vi "Dresden R2R Sputter 03.02.2018 IY24.vi"() -> ()   [LabVIEW 2009] (continued)
                                frame #0 {
                                n26763 = while {
                                i -> [w31945]
                                stop <- w31941 stop-if-true
                                n26764 = local read "Pc_bv_opened_ch3"() -> (w31943:bool)
                                n26765 = Greater?(x=w31945, y=120) -> (0:w31944:bool)
                                n26766 = local read "Semi"() -> (w31942:bool)
                                n26767 = Compound Arithmetic op=OR(w31942, w31943, w31944) -> (w31941:bool)
                                n26768 = Wait (ms)(milliseconds to wait=u32 500) -> ()  [unwired: 1 out]
                                }
                                }
                                frame #1 {
                                }
                                }
                                }
                                frame #6 {
                                n26769 = local read "Semi"() -> (w31947:bool)
                                n26770 = case shown="False" w31947 {
                                frame #0 {
                                n26771 = local read "Pc_bv_opened_ch3"() -> (w31948:bool)
                                n26772 = case shown="False" w31948 {
                                frame #0 {
                                n26773 = local write "Error Message"("Start up process  cancelled\nbecause  PC-BV not opened.\nPlease check PC-BV1 connections." ("Error Message")) -> ()
                                n26774 = Wait (ms)(milliseconds to wait=u32 1000) -> ()  [unwired: 1 out]
                                }
                                frame #1 {
                                }
                                }
                                }
                                frame #1 {
                                }
                                }
                                }
                                }
                                }
                                frame #1 {
                                }
                                }
                                }
                                frame #1 {
                                n26775 = local read "Semi"() -> (w31951:bool)
                                n26776 = case shown="False" w31951 {
                                frame #0 {
                                n26777 = Wait (ms)(milliseconds to wait=u32 1000) -> ()  [unwired: 1 out]
                                n26778 = local write "SDC1 7"(TRUE ("SDC1 7")) -> ()
                                }
                                frame #1 {
                                }
                                }
                                }
                                }
                                }
                                frame #10 {
                                # "CC OPEN"
                                n26779 = stacked-sequence {
                                frame #0 {
                                n26780 = local read "Semi"() -> (w31954:bool)
                                n26781 = case shown="False" w31954 {
                                frame #0 {
                                n26782 = while {
                                i -> [w31960]
                                stop <- w31955 stop-if-true
                                n26783 = Greater?(x=w31960, y=50) -> (0:w31959:bool)
                                n26784 = case shown="True" w31959 {
                                frame #0 {
                                }
                                frame #1 {
                                n26785 = local write "Semi"(TRUE ("Semi")) -> ()
                                n26786 = local write "Error Message"("Coating Process  \nwas cancelled.\nPlease check \nBG-BV connection." ("Error Message")) -> ()
                                }
                                }
                                n26787 = local read "Ch3_Cc_on_off_di"() -> (w31958:bool)
                                n26788 = case shown="False" w31958 {
                                tunnel: [FALSE TRUE] -> w31957
                                frame #0 {
                                n26789 = local write "Ch3_Cc_on_off_do"(TRUE ("Ch1_WFC_do")) -> ()
                                n26790 = Wait Until Next ms Multiple(millisecond multiple=u32 200) -> ()  [unwired: 1 out]
                                }
                                frame #1 {
                                }
                                }
                                n26791 = local read "Semi"() -> (w31956:bool)
                                n26792 = Or(x=w31957, y=w31956) -> (x .or. y?=w31955:bool)
                                }
                                }
                                frame #1 {
                                }
                                }
                                }
                                frame #1 {
                                n26793 = local read "Semi"() -> (w31968:bool)
                                n26794 = case shown="False" w31968 {
                                frame #0 {
                                n26795 = while {
                                i -> [w31973]
                                stop <- w31971 stop-if-true
                                n26796 = Greater?(x=w31973, y=30) -> (0:w31969:bool)
                                n26797 = Wait Until Next ms Multiple(millisecond multiple=u32 1000) -> ()  [unwired: 1 out]
                                n26798 = local read "Semi"() -> (w31972:bool)
                                n26799 = Or(x=w31969, y=w31972) -> (x .or. y?=w31971:bool)
                                }
                                }
                                frame #1 {
                                }
                                }
                                }
                                frame #2 {
                                n26800 = local read "Semi"() -> (w31975:bool)
                                n26801 = case shown="False" w31975 {
                                frame #0 {
                                n26802 = Wait (ms)(milliseconds to wait=u32 1000) -> ()  [unwired: 1 out]
                                n26803 = local write "SDC1 7b"(TRUE ("SDC1 3")) -> ()
                                }
                                frame #1 {
                                }
                                }
                                }
                                }
                                }
                                frame #11 {
                                # "CHECK CHAMBER PRESSURE"
                                n26804 = stacked-sequence {
                                frame #0 {
                                n26805 = local read "Semi"() -> (w31978:bool)
                                n26806 = case shown="False" w31978 {
                                frame #0 {
                                n26807 = while {
                                i -> [w31986]
                                stop <- w31980 stop-if-true
                                n26808 = Greater?(x=w31986, y=300) -> (0:w31985:bool)
                                n26809 = case shown="True" w31985 {
                                frame #0 {
                                }
                                frame #1 {
                                n26810 = local write "Semi"(TRUE ("Semi")) -> ()
                                n26811 = local write "Error Message"("Coating Process cancelled.\nPlease check chamber \nconnections." ("Error Message")) -> ()
                                }
                                }
                                n26812 = local read "Ch_CC_press_ch3 2"() -> (w31979:dbl)
                                n26813 = Greater Or Equal?(x=w31979, y=5e-05 ("CHAMBER PRESSURE 5")) -> (x >= y?=w31983:bool)
                                n26814 = case shown="True" w31983 {
                                tunnel: [TRUE FALSE] -> w31982
                                frame #0 {
                                }
                                frame #1 {
                                n26815 = Wait Until Next ms Multiple(millisecond multiple=u32 200) -> ()  [unwired: 1 out]
                                }
                                }
                                n26816 = local read "Semi"() -> (w31981:bool)
                                n26817 = Or(x=w31982, y=w31981) -> (x .or. y?=w31980:bool)
                                }
                                }
                                frame #1 {
                                }
                                }
                                }
                                frame #1 {
                                n26818 = local read "Semi"() -> (w31993:bool)
                                n26819 = case shown="False" w31993 {
                                frame #0 {
                                n26820 = Wait (ms)(milliseconds to wait=u32 1000) -> ()  [unwired: 1 out]
                                n26821 = local write "SDC1 10"(TRUE ("SDC1 10")) -> ()
                                }
                                frame #1 {
                                }
                                }
                                }
                                }
                                }
                                frame #12 {
                                # "CC CLOSE"
                                n26822 = stacked-sequence {
                                frame #0 {
                                n26823 = local read "Semi"() -> (w31996:bool)
                                n26824 = case shown="False" w31996 {
                                frame #0 {
                                n26825 = while {
                                i -> [w32002]
                                stop <- w31997 stop-if-true
                                n26826 = Greater?(x=w32002, y=50) -> (0:w32001:bool)
                                n26827 = case shown="True" w32001 {
                                frame #0 {
                                }
                                frame #1 {
                                n26828 = local write "Semi"(TRUE ("Semi")) -> ()
                                n26829 = local write "Error Message"("Coating Process  \nwas cancelled.\nPlease check \nBG-BV connection." ("Error Message")) -> ()
                                }
                                }
                                n26830 = local read "Ch3_Cc_on_off_di"() -> (w32000:bool)
                                n26831 = case shown="True" w32000 {
                                tunnel: [TRUE FALSE] -> w31999
                                frame #0 {
                                }
                                frame #1 {
                                n26832 = local write "Ch3_Cc_on_off_do"(FALSE ("Ch1_WFC_do")) -> ()
                                n26833 = Wait Until Next ms Multiple(millisecond multiple=u32 200) -> ()  [unwired: 1 out]
                                }
                                }
                                n26834 = local read "Semi"() -> (w31998:bool)
                                n26835 = Or(x=w31999, y=w31998) -> (x .or. y?=w31997:bool)
                                }
                                }
                                frame #1 {
                                }
                                }
                                }
                                frame #1 {
                                n26836 = local read "Semi"() -> (w32010:bool)
                                n26837 = case shown="False" w32010 {
                                frame #0 {
                                n26838 = local write "SDC1 10b"(TRUE ("SDC1 3")) -> ()
                                n26839 = Wait (ms)(milliseconds to wait=u32 1000) -> ()  [unwired: 1 out]
                                }
                                frame #1 {
                                }
                                }
                                }
                                }
                                }
                                frame #13 {
                                # "SET Ar FLOW"
                                n26840 = local read "R_Web_selection"() -> (w32013:enum32{"Web", "Other"})
                                n26841 = case shown="\"Other\"" w32013 {
                                frame #0 {
                                }
                                frame #1 {
                                n26842 = stacked-sequence {
                                frame #0 {
                                n26843 = local read "Semi"() -> (w32014:bool)
                                n26844 = case shown="False" w32014 {
                                frame #0 {
                                n26845 = stacked-sequence {
                                frame #0 {
                                n26846 = local read "Semi"() -> (w32015:bool)
                                n26847 = case shown="False" w32015 {
                                frame #0 {
                                n26848 = local read "R Argon Flow sccm"() -> (w32016:dbl)
                                n26849 = local write "Ar_sccm3_4"(w32016) -> ()
                                }
                                frame #1 {
                                }
                                }
                                }
                                frame #1 {
                                n26850 = local read "Semi"() -> (w32017:bool)
                                n26851 = case shown="False" w32017 {
                                frame #0 {
                                n26852 = local write "Mfc2_Ar _3_4_set"(TRUE ("Mfc_Ar _1_2_set")) -> ()
                                }
                                frame #1 {
                                }
                                }
                                }
                                frame #2 {
                                n26853 = local read "Semi"() -> (w32019:bool)
                                n26854 = case shown="False" w32019 {
                                frame #0 {
                                n26855 = while {
                                i -> [w32022]
                                stop <- w32024 stop-if-true
                                n26856 = Greater?(x=w32022, y=50) -> (0:w32021:bool)
                                n26857 = local read "Semi"() -> (w32020:bool)
                                n26858 = Or(x=w32020, y=w32021) -> (x .or. y?=w32024:bool)
                                }
                                }
                                frame #1 {
                                }
                                }
                                }
                                frame #3 {
                                n26859 = local read "Semi"() -> (w32025:bool)
                                n26860 = case shown="False" w32025 {
                                frame #0 {
                                n26861 = local read "Ar_sccm_act 2"() -> (w32026:dbl)
                                n26862 = Greater?(x=w32026, y=1) -> (0:w32027:bool)
                                n26863 = case shown="False" w32027 {
                                frame #0 {
                                n26864 = local read "R Argon Flow sccm"() -> (w32029:dbl)
                                n26865 = local write "Ar_sccm3_4"(w32029) -> ()
                                }
                                frame #1 {
                                }
                                }
                                }
                                frame #1 {
                                }
                                }
                                }
                                frame #4 {
                                n26866 = local read "Semi"() -> (w32030:bool)
                                n26867 = case shown="False" w32030 {
                                frame #0 {
                                n26868 = local read "Ar_sccm_act 2"() -> (w32031:dbl)
                                n26869 = Greater?(x=w32031, y=1) -> (0:w32032:bool)
                                n26870 = case shown="False" w32032 {
                                frame #0 {
                                n26871 = while {
                                i -> [w32035]
                                stop <- w32039 stop-if-true
                                n26872 = Greater?(x=w32035, y=50) -> (0:w32034:bool)
                                n26873 = local read "Semi"() -> (w32038:bool)
                                n26874 = case shown="False" w32038 {
                                tunnel: [FALSE TRUE] -> w32037
                                frame #0 {
                                n26875 = Wait Until Next ms Multiple(millisecond multiple=u32 200) -> ()  [unwired: 1 out]
                                }
                                frame #1 {
                                }
                                }
                                n26876 = Or(x=w32037, y=w32034) -> (x .or. y?=w32039:bool)
                                }
                                }
                                frame #1 {
                                }
                                }
                                }
                                frame #1 {
                                }
                                }
                                }
                                frame #5 {
                                n26877 = local read "Semi"() -> (w32043:bool)
                                n26878 = case shown="False" w32043 {
                                frame #0 {
                                n26879 = local read "Ar_sccm_act 2"() -> (w32044:dbl)
                                n26880 = Greater?(x=w32044, y=1) -> (0:w32045:bool)
                                n26881 = case shown="False" w32045 {
                                frame #0 {
                                n26882 = local write "Semi"(TRUE ("Semi")) -> ()
                                n26883 = local write "Error Message"("Coating process cancelled.\nPlease check connections." ("Error Message")) -> ()
                                }
                                frame #1 {
                                }
                                }
                                }
                                frame #1 {
                                }
                                }
                                }
                                }
                                }
                                frame #1 {
                                }
                                }
                                }
                                frame #1 {
                                n26884 = local read "Semi"() -> (w32049:bool)
                                n26885 = case shown="False" w32049 {
                                frame #0 {
                                n26886 = local write "SDC1 11"(TRUE ("SDC1 11")) -> ()
                                n26887 = Wait (ms)(milliseconds to wait=u32 1000) -> ()  [unwired: 1 out]
                                }
                                frame #1 {
                                }
                                }
                                }
                                }
                                }
                                }
                                }
                                frame #14 {
                                # "Set  Pressure"
                                n26888 = local read "R_Web_selection"() -> (w32052:enum32{"Web", "Other"})
                                n26889 = case shown="\"Other\"" w32052 {
                                frame #0 {
                                }
                                frame #1 {
                                n26890 = stacked-sequence {
                                frame #0 {
                                n26891 = local read "Semi"() -> (w32053:bool)
                                n26892 = case shown="False" w32053 {
                                frame #0 {
                                n26893 = stacked-sequence {
                                frame #0 {
                                n26894 = local read "Semi"() -> (w32054:bool)
                                n26895 = case shown="False" w32054 {
                                frame #0 {
                                n26896 = local read "R Set Pressure mtorr"() -> (w32055:dbl)
                                n26897 = local write "Set_pressure_value 3"(w32055) -> ()
                                }
                                frame #1 {
                                }
                                }
                                }
                                frame #1 {
                                n26898 = local read "Semi"() -> (w32056:bool)
                                n26899 = case shown="False" w32056 {
                                frame #0 {
                                n26900 = Wait (ms)(milliseconds to wait=u32 1000) -> ()  [unwired: 1 out]
                                }
                                frame #1 {
                                }
                                }
                                }
                                frame #2 {
                                n26901 = local read "Semi"() -> (w32058:bool)
                                n26902 = case shown="False" w32058 {
                                frame #0 {
                                n26903 = local write "Pc_bv3_auto_set_pressure"(TRUE ("Pc_bv1_auto_set_pressure")) -> ()
                                }
                                frame #1 {
                                }
                                }
                                }
                                frame #3 {
                                n26904 = local read "Semi"() -> (w32060:bool)
                                n26905 = case shown="False" w32060 {
                                frame #0 {
                                n26906 = while {
                                i -> [w32071]
                                stop <- w32063 stop-if-true
                                n26907 = Greater?(x=w32071, y=300) -> (0:w32065:bool)
                                n26908 = local read "Set_pressure_value 3"() -> (w32061:dbl)
                                n26909 = Add(x=1.0, y=w32061) -> (x+y=w32067:dbl)
                                n26910 = Subtract(x=w32061, y=1.0) -> (x-y=w32068:dbl)
                                n26911 = local read "Pressure_ch3"() -> (w32062:i32)
                                n26912 = In Range and Coerce(upper limit=w32067, x=w32062, lower limit=w32068) -> (In Range?=w32066:bool)  [unwired: 1 out]
                                n26913 = case shown="False" w32066 {
                                tunnel: [FALSE TRUE] -> w32064
                                frame #0 {
                                n26914 = Wait Until Next ms Multiple(millisecond multiple=u32 200) -> ()  [unwired: 1 out]
                                }
                                frame #1 {
                                }
                                }
                                n26915 = Or(x=w32064, y=w32065) -> (x .or. y?=w32063:bool)
                                }
                                }
                                frame #1 {
                                }
                                }
                                }
                                frame #4 {
                                n26916 = local read "Semi"() -> (w32076:bool)
                                n26917 = case shown="False" w32076 {
                                frame #0 {
                                n26918 = local read "Set_pressure_value 3"() -> (w32078:dbl)
                                n26919 = Add(x=1.0, y=w32078) -> (x+y=w32080:dbl)
                                n26920 = Subtract(x=w32078, y=1.0) -> (x-y=w32081:dbl)
                                n26921 = local read "Pressure_ch3"() -> (w32077:i32)
                                n26922 = In Range and Coerce(upper limit=w32080, x=w32077, lower limit=w32081) -> (In Range?=w32079:bool)  [unwired: 1 out]
                                n26923 = case shown="False" w32079 {
                                frame #0 {
                                n26924 = local read "R Set Pressure mtorr"() -> (w32084:dbl)
                                n26925 = local write "Set_pressure_value 3"(w32084) -> ()
                                }
                                frame #1 {
                                }
                                }
                                }
                                frame #1 {
                                }
                                }
                                }
                                frame #5 {
                                n26926 = local read "Semi"() -> (w32085:bool)
                                n26927 = case shown="False" w32085 {
                                frame #0 {
                                n26928 = local read "Set_pressure_value 3"() -> (w32087:dbl)
                                n26929 = Add(x=1.0, y=w32087) -> (x+y=w32089:dbl)
                                n26930 = Subtract(x=w32087, y=1.0) -> (x-y=w32090:dbl)
                                n26931 = local read "Pressure_ch3"() -> (w32086:i32)
                                n26932 = In Range and Coerce(upper limit=w32089, x=w32086, lower limit=w32090) -> (In Range?=w32088:bool)  [unwired: 1 out]
                                n26933 = case shown="False" w32088 {
                                frame #0 {
                                n26934 = local write "Pc_bv3_auto_set_pressure"(TRUE ("Pc_bv1_auto_set_pressure")) -> ()
                                }
                                frame #1 {
                                }
                                }
                                }
                                frame #1 {
                                }
                                }
                                }
                                frame #6 {
                                n26935 = local read "Semi"() -> (w32094:bool)
                                n26936 = case shown="False" w32094 {
                                frame #0 {
                                n26937 = while {
                                i -> [w32105]
                                stop <- w32097 stop-if-true
                                n26938 = Greater?(x=w32105, y=300) -> (0:w32099:bool)
                                n26939 = local read "Set_pressure_value 3"() -> (w32096:dbl)
                                n26940 = Add(x=1.0, y=w32096) -> (x+y=w32101:dbl)
                                n26941 = Subtract(x=w32096, y=1.0) -> (x-y=w32102:dbl)
                                n26942 = local read "Pressure_ch3"() -> (w32095:i32)
                                n26943 = In Range and Coerce(upper limit=w32101, x=w32095, lower limit=w32102) -> (In Range?=w32100:bool)  [unwired: 1 out]
                                n26944 = case shown="False" w32100 {
                                tunnel: [FALSE TRUE] -> w32098
                                frame #0 {
                                n26945 = Wait Until Next ms Multiple(millisecond multiple=u32 200) -> ()  [unwired: 1 out]
                                }
                                frame #1 {
                                }
                                }
                                n26946 = Or(x=w32098, y=w32099) -> (x .or. y?=w32097:bool)
                                }
                                }
                                frame #1 {
                                }
                                }
                                }
                                frame #7 {
                                n26947 = local read "Semi"() -> (w32110:bool)
                                n26948 = case shown="False" w32110 {
                                frame #0 {
                                n26949 = local read "Set_pressure_value 3"() -> (w32112:dbl)
                                n26950 = Add(x=1.0, y=w32112) -> (x+y=w32114:dbl)
                                n26951 = Subtract(x=w32112, y=1.0) -> (x-y=w32115:dbl)
                                n26952 = local read "Pressure_ch3"() -> (w32111:i32)
                                n26953 = In Range and Coerce(upper limit=w32114, x=w32111, lower limit=w32115) -> (In Range?=w32113:bool)  [unwired: 1 out]
                                n26954 = case shown="False" w32113 {
                                frame #0 {
                                n26955 = local write "Semi"(TRUE ("Semi")) -> ()
                                n26956 = local write "Error Message"("Coating Pressure could not be adjusted !" ("Error Message")) -> ()
                                }
                                frame #1 {
                                }
                                }
                                }
                                frame #1 {
                                }
                                }
                                }
                                }
                                }
                                frame #1 {
                                }
                                }
                                }
                                frame #1 {
                                n26957 = local read "Semi"() -> (w32120:bool)
                                n26958 = case shown="False" w32120 {
                                frame #0 {
                                n26959 = local write "SDC1 9"(TRUE ("SDC1 9")) -> ()
                                n26960 = Wait (ms)(milliseconds to wait=u32 1000) -> ()  [unwired: 1 out]
                                }
                                frame #1 {
                                }
                                }
                                }
                                }
                                }
                                }
                                }
                                frame #15 {
                                # "DC -Ignite Plasma"
                                n26961 = stacked-sequence {
                                frame #0 {
                                n26962 = local read "Semi"() -> (w32123:bool)
                                n26963 = case shown="False" w32123 {
                                frame #0 {
                                n26964 = stacked-sequence {
                                frame #0 {
                                n26965 = local read "Semi"() -> (w32124:bool)
                                n26966 = case shown="False" w32124 {
                                frame #0 {
                                n26967 = while {
                                i -> [w32130]
                                stop <- w32125 stop-if-true
                                n26968 = Greater?(x=w32130, y=50) -> (0:w32129:bool)
                                n26969 = case shown="True" w32129 {
                                frame #0 {
                                }
                                frame #1 {
                                n26970 = local write "Semi"(TRUE ("Semi")) -> ()
                                n26971 = local write "Error Message"("Sputtering Process cancelled.\nPlease check \nDC switch connections." ("Error Message")) -> ()
                                }
                                }
                                n26972 = local read "Cnt_Dcps_sw2_di"() -> (w32128:bool)
                                n26973 = case shown="False" w32128 {
                                tunnel: [FALSE ("Cnt_Dcps_sw1_do") TRUE ("Cnt_Dcps_sw1_do")] -> w32127
                                frame #0 {
                                n26974 = local write "Cnt_Dcps_sw2_do"(TRUE ("Cnt_Dcps_sw1_do")) -> ()
                                n26975 = Wait Until Next ms Multiple(millisecond multiple=u32 200) -> ()  [unwired: 1 out]
                                }
                                frame #1 {
                                }
                                }
                                n26976 = local read "Semi"() -> (w32126:bool)
                                n26977 = Or(x=w32127, y=w32126) -> (x .or. y?=w32125:bool)
                                }
                                }
                                frame #1 {
                                }
                                }
                                }
                                frame #1 {
                                n26978 = local read "Semi"() -> (w32138:bool)
                                n26979 = case shown="False" w32138 {
                                frame #0 {
                                n26980 = while {
                                i -> [w32144]
                                stop <- w32139 stop-if-true
                                n26981 = Greater?(x=w32144, y=50) -> (0:w32143:bool)
                                n26982 = case shown="True" w32143 {
                                frame #0 {
                                }
                                frame #1 {
                                n26983 = local write "Semi"(TRUE ("Semi")) -> ()
                                n26984 = local write "Error Message"("Sputtering Process cancelled.\nPlease check \nDC switch connections." ("Error Message")) -> ()
                                }
                                }
                                n26985 = local read "Cnt_Dcps_sw1_di"() -> (w32142:bool)
                                n26986 = case shown="True" w32142 {
                                tunnel: [TRUE ("Cnt_Dcps_sw1_do") FALSE ("Cnt_Dcps_sw1_do")] -> w32141
                                frame #0 {
                                }
                                frame #1 {
                                n26987 = local write "Cnt_Dcps_sw1_do"(FALSE ("Cnt_Dcps_sw1_do")) -> ()
                                n26988 = Wait Until Next ms Multiple(millisecond multiple=u32 200) -> ()  [unwired: 1 out]
                                }
                                }
                                n26989 = local read "Semi"() -> (w32140:bool)
                                n26990 = Or(x=w32141, y=w32140) -> (x .or. y?=w32139:bool)
                                }
                                }
                                frame #1 {
                                }
                                }
                                }
                                frame #2 {
                                n26991 = local read "Semi"() -> (w32152:bool)
                                n26992 = case shown="False" w32152 {
                                frame #0 {
                                n26993 = local write "Dc_host_auto"(TRUE ("Dc_host_auto")) -> ()
                                }
                                frame #1 {
                                }
                                }
                                }
                                frame #3 {
                                n26994 = local read "Semi"() -> (w32154:bool)
                                n26995 = case shown="False" w32154 {
                                frame #0 {
                                n26996 = local read "R Single DC Step1 Coating Power"() -> (w32155:dbl)
                                n26997 = local write "Set DC Power       : 2"(w32155) -> ()
                                }
                                frame #1 {
                                }
                                }
                                }
                                frame #4 {
                                n26998 = local read "Semi"() -> (w32156:bool)
                                n26999 = case shown="False" w32156 {
                                frame #0 {
                                n27000 = Wait (ms)(milliseconds to wait=u32 1000) -> ()  [unwired: 1 out]
                                }
                                frame #1 {
                                }
                                }
                                }
                                frame #5 {
                                n27001 = local read "Semi"() -> (w32158:bool)
                                n27002 = case shown="False" w32158 {
                                frame #0 {
                                n27003 = local write "Dc_auto_set"(TRUE ("Dc_auto_set")) -> ()
                                }
                                frame #1 {
                                }
                                }
                                }
                                frame #6 {
                                n27004 = Wait (ms)(milliseconds to wait=u32 1000) -> ()  [unwired: 1 out]
                                }
                                frame #7 {
                                n27005 = local read "Semi"() -> (w32161:bool)
                                n27006 = case shown="False" w32161 {
                                frame #0 {
                                n27007 = local read "Web_selection_tab"() -> (w32162:T5)
                                n27008 = case shown="\"Other                                                                                    \"" w32162 {
                                frame #0 {
                                }
                                frame #1 {
                                n27009 = local write "Dc_auto_on"(TRUE ("Dc_auto_on")) -> ()
                                }
                                }
                                }
                                frame #1 {
                                }
                                }
                                }
                                frame #8 {
                                n27010 = local read "Web_selection_tab"() -> (w32164:T5)
                                n27011 = case shown="\"Other                                                                                    \"" w32164 {
                                frame #0 {
                                }
                                frame #1 {
                                n27012 = local read "Semi"() -> (w32165:bool)
                                n27013 = case shown="False" w32165 {
                                frame #0 {
                                n27014 = while {
                                i -> [w32175]
                                stop <- w32168 stop-if-true
                                n27015 = Greater Or Equal?(x=w32175, y=240) -> (x >= y?=w32174:bool)
                                n27016 = case shown="True" w32174 {
                                frame #0 {
                                }
                                frame #1 {
                                n27017 = local write "Semi"(TRUE ("Semi")) -> ()
                                }
                                }
                                n27018 = local read "Actual DC Power : 2"() -> (w32166:dbl)
                                n27019 = local read "Set DC Power       : 2"() -> (w32167:dbl)
                                n27020 = Subtract(x=w32167, y=w32166) -> (x-y=w32173:dbl)
                                n27021 = Less?(x=w32173, y=10.0) -> (x < y?=w32170:bool)
                                n27022 = local read "Semi"() -> (w32169:bool)
                                n27023 = Or(x=w32170, y=w32169) -> (x .or. y?=w32168:bool)
                                n27024 = Wait Until Next ms Multiple(millisecond multiple=u32 500) -> ()  [unwired: 1 out]
                                }
                                }
                                frame #1 {
                                }
                                }
                                }
                                }
                                }
                                frame #9 {
                                n27025 = local read "Semi"() -> (w32178:bool)
                                n27026 = case shown="False" w32178 {
                                frame #0 {
                                n27027 = Wait (ms)(milliseconds to wait=u32 1000) -> ()  [unwired: 1 out]
                                }
                                frame #1 {
                                }
                                }
                                }
                                }
                                }
                                frame #1 {
                                }
                                }
                                }
                                frame #1 {
                                n27028 = local read "Semi"() -> (w32180:bool)
                                n27029 = case shown="False" w32180 {
                                frame #0 {
                                n27030 = Wait (ms)(milliseconds to wait=u32 1000) -> ()  [unwired: 1 out]
                                n27031 = local write "SDC1 13"(TRUE ("SDC1 13")) -> ()
                                }
                                frame #1 {
                                }
                                }
                                }
                                }
                                }
                                frame #16 {
                                n27032 = local read "Web_selection_tab"() -> (w32183:T5)
                                n27033 = case shown="\"Web                                                                                    \", Default" w32183 {
                                frame #0 {
                                n27034 = stacked-sequence {
                                frame #0 {
                                n27035 = local read "R Maximum diameter"() -> (w32185:dbl)
                                n27036 = local read "R Web speed(cm/min)"() -> (w32187:dbl)
                                n27037 = local read "R Minimum diameter"() -> (w32184:dbl)
                                n27038 = local read "R Web thicness"() -> (w32186:dbl)
                                n27039 = Wait (ms)(milliseconds to wait=u32 100) -> ()  [unwired: 1 out]
                                n27040 = local write "Initial Min Diameter"(w32184) -> ()
                                n27041 = local write "Max Diameter"(w32185) -> ()
                                n27042 = local write "Web Thickness"(w32186) -> ()
                                n27043 = local write "Web Speed"(w32187) -> ()
                                }
                                frame #1 {
                                n27044 = local read "R Single DC Step1 Coating Power Active"() -> (w32202:bool)
                                n27045 = local read "R Single DC Step2 Coating Power Active"() -> (w32201:bool)
                                n27046 = local read "R Single DC Step3 Coating Power Active"() -> (w32200:bool)
                                n27047 = local read "R Single DC Step4 Coating Power Active"() -> (w32199:bool)
                                n27048 = local read "R Single DC Step5 Coating Power Active"() -> (w32198:bool)
                                n27049 = Boolean To (0,1)(Boolean=w32202) -> (0, 1=w32197:i16)
                                n27050 = Boolean To (0,1)(Boolean=w32201) -> (0, 1=w32196:i16)
                                n27051 = Boolean To (0,1)(Boolean=w32200) -> (0, 1=w32195:i16)
                                n27052 = Boolean To (0,1)(Boolean=w32199) -> (0, 1=w32194:i16)
                                n27053 = Boolean To (0,1)(Boolean=w32198) -> (0, 1=w32193:i16)
                                n27054 = Compound Arithmetic op=ADD(w32197, w32196, w32195, w32194, w32193) -> (w32191:i16)
                                n27055 = local read "R Single DC Interval length"() -> (w32192:dbl)
                                n27056 = Wait (ms)(milliseconds to wait=u32 200) -> ()  [unwired: 1 out]
                                n27057 = Multiply(x=w32192, y=w32191) -> (x*y=w32190:dbl)
                                n27058 = local write "Total length"(w32190) -> ()
                                }
                                frame #2 {
                                n27059 = local write "Calculate 2"(TRUE ("Calculate_auto")) -> ()
                                }
                                frame #3 {
                                n27060 = local write "Roll_side_select"(enum32{"Left to Right", "Right to Left"}."Left to Right" ("Roll_side_select")) -> ()